vi "AbsImage_LFHelper_PIXIS_v0.1.vi"() -> ()   [LabVIEW 2012]
doc: "Take a single PixelFly exposure and display the result as an intensity graph.This VI illustrates the basics of taking an exposure with the PixelFly camera. Use Ctrl-H to get help on any of the controls\n\nCopyright 2001, The Cooke Corporation."
uses:
  LabVIEW Data V4.10/Shared Libraries/Controls/FileName_Cluster.ctl
  IMAQdx_AbsImage_Flea3_v4.2_RbYb/Shared Libraries/Controls/FileInfo_Global.vi
  <vilib>/Analysis/NI_AALBase.lvlib
panel:
  out "CycleDone":bool
  out "frame count":i64
  out "Loop":i32=3
  out "Status":string="Running..."
  in  "stop":bool
  in  "Tab Control":enum32{"Setup", "Images", "Hardware status"}(tab)=enum."Images"
  in  "SPE File Path":path=path "C:/Users/Lab/Documents/LightField/LabviewTemp.spe"
  in  "Experiment":T1(ring)=enum."Sr"
  in  "Accept parameters from remote system":bool=TRUE
  in  "Bias (Amps)":dbl
  in  "Pinch Coil (Amps)":dbl=520.0
  in  "Expansion time (ms)":dbl=19.0
  in  "Trap min at 0 (MHz)":dbl=2.85
  in  "Detuning (Linewidths)":dbl
  in  "Racetrack (Amps)":dbl=540.0
  in  "Magnification":dbl=5.66
  in  "Image direction":enum16{"XY", "XZ"}(ring)
  in  "Imaging technique":enum16{"Absorption", "Fluorescence", "RawImage"}(ring)
  in  "File Parameters":T2={"Data Root"=path "C:/Experiment/Data", "Index"=20198, "Instrument"="PIXIS"} {"Index" format="%04d"}
  in  "Send data to Igor?":bool=TRUE
  out "Command to Igor":string="AutoRunV3(\"Dipole_Load_Sr_88\",\"C:\\\\Experiment\\\\Data\\\\2013\\\\October\\\\09\\\\PIXIS_09Oct2013_20197.ibw\") "
  out "Image note":string="Experiment=Sr\nCamera_ID=PIXIS\nImageType=Raw\nDataType=Absorption\nImageDirection=XY\nMagnification=5.660000E+0\nFileNumber=20197\n# Current Variables\n# \nplus_zman=-1.800000E+0\nminus_zman=-1.500000E+0\ncompensation=-1.500000E+0\nMOTcoils=-1.250000E+0\nx=1.000000E+0\n# Master Staging List\n# Line\tMarker\tOption\tHalt\t0       4       8      12      16      20    AO\tDelay\t\tPoints\t0\t\t1\t\t2\t\t3\t\t4\t\t5\t\t6\t\t7\t\t8\t\t9\t\t10\t\t11\t\t12\t\t13\t\t14\t\t15\t\tComment\n00\t\tRamp\t0 0 0 0 0 0 0 0 0 0 1 0 0 1 0 0 0 0 0 0 0 0 0 0\t.5\t0\tplus_zman\tminus_zman\tcompensation\tMOTcoils\t0\t0\t0\t0\t0\t0\t0\t0\t0\t0\t0\t0\twait\n01\t\tRamp\t0 0 0 0 0 0 0 0 0 0 1 0 0 1 0 0 0 0 0 0 0 0 0 0\t.0001\t0\tplus_zman\tminus_zman\tcompensation\tMOTcoils\t0\t0\t0\t0\t0\t0\t0\t0\tLineRamp(f, 2,10)\t0\t0\t0\timg 1\n02\t\tRamp\t0 0 0 0 0 0 0 0 0 0 1 0 0 1 0 0 0 0 0 0 0 0 0 0\t.75\t0\tplus_zman\tminus_zman\tcompensation\tMOTcoils\t0\t0\t0\t0\t0\t0\t0\t0\t5\t0\t0\t0\ttransmit\n03\t\tRamp\t0 0 0 0 0 0 0 0 0 0 1 0 0 1 0 0 0 0 0 0 0 0 0 0\t.0001\t0\tplus_zman\tminus_zman\tcompensation\tMOTcoils\t0\t0\t0\t0\t0\t0\t0\t0\tSinRamp(t,5,2,5,0)\t0\t0\t0\timg 2\n04\t\tRamp\t0 0 0 0 0 0 0 0 0 0 1 0 0 1 0 0 0 0 0 0 0 0 0 0\t.75\t0\tplus_zman\tminus_zman\tcompensation\tMOTcoils\t0\t0\t0\t0\t0\t0\t0\t0\t0\t0\t0\t0\ttransmit\n05\t\tRamp\t0 0 0 0 0 0 0 0 0 0 1 0 0 1 0 0 0 0 0 0 0 0 0 0\t.0001\t0\t-1.8\t-1.5\t-1.5\t-1.25\t0\t0\t0\t0\t0\t0\t0\t0\t0\t0\t0\t0\timg 3\n06\t\tRamp\t0 0 0 0 0 0 0 0 0 0 1 0 0 1 0 0 0 0 0 0 0 0 0 0\t.75\t0\t-1.8\t-1.5\t-1.5\t-1.25\t0\t0\t0\t0\t0\t0\t0\t0\t0\t0\t0\t0\ttransmit\n07\t\tRamp\t0 0 0 0 0 0 0 0 0 0 1 0 0 1 0 0 0 0 0 0 0 0 0 0\t.0001\t0\t-1.8\t-1.5\t-1.5\t-1.25\t0\t0\t0\t0\t0\t0\t0\t0\t0\t0\t0\t0\timg 4\n08\t\tRamp\t0 0 0 0 0 0 0 0 0 0 1 0 0 1 0 0 0 0 0 0 0 0 0 0\t.75\t0\t-1.8\t-1.5\t-1.5\t-1.25\t0\t0\t0\t0\t0\t0\t0\t0\t0\t0\t0\t0\ttransmit\n# Slave Staging List\n# Line\tMarker\tOption\tHalt\t0       4       8      12      16      20    AO\tDelay\t\tPoints\t0\t\t1\t\t2\t\t3\t\t4\t\t5\t\t6\t\t7\t\t8\t\t9\t\t10\t\t11\t\t12\t\t13\t\t14\t\t15\t\tComment\n# SRS List\n# \n#\n# Evaporation\n\nDDS Table\r\n"
  in  "Igor Wave Name":string="Test_Img"
  in  "Save file to archive?":bool=TRUE
  in  "Quad [Amps]":dbl=540.0
  in  "Source of File Data":refnum<k21>="\\\\Control\\VariableLibrary\\Instruction String"
  in  "Bits to shift":i32
  out "SPE delete path":path=path "C:/Users/Lab/Documents/LightField/LabviewTemp.spe"
  in  "Source of Control Data":refnum<k21>="\\\\CONTROL\\VariableLibrary\\CycleDone"
  in  "Raw image to view":u16(ring)=3 items=["Clear", "Absorbtion", "Probe", "Background"]
  in  "Update Graphics":bool=TRUE
  out "Raw Image":u16[][](graph)
  out "Processed Image":sgl[][](graph)
  out "Histogram":cluster{"X Values":dbl[], dbl[]}(graph)={"X Values"=[222.6796875, 228.0390625, 233.3984375, 238.7578125, 244.1171875, 249.4765625, 254.8359375, 260.1953125, 265.5546875, 270.9140625, 276.2734375, 281.6328125, 286.9921875, 292.3515625, 297.7109375, 303.0703125, 308.4296875, 313.7890625, 319.1484375, 324.5078125, 329.8671875, 335.2265625, 340.5859375, 345.9453125, 351.3046875, 356.6640625, 362.0234375, 367.3828125, 372.7421875, 378.1015625, 383.4609375, 388.8203125, 394.1796875, 399.5390625, 404.8984375, 410.2578125, 415.6171875, 420.9765625, 426.3359375, 431.6953125, 437.0546875, 442.4140625, 447.7734375, 453.1328125, 458.4921875, 463.8515625, 469.2109375, 474.5703125, 479.9296875, 485.2890625, 490.6484375, 496.0078125, 501.3671875, 506.7265625, 512.0859375, 517.4453125, 522.8046875, 528.1640625, 533.5234375, 538.8828125, 544.2421875, 549.6015625, 554.9609375, 560.3203125], [0.0, 0.0, 0.47712125471966244, 0.9030899869919435, 1.3979400086720377, 1.7558748556724915, 1.9084850188786497, 2.0827853703164503, 2.2764618041732443, 2.250420002308894, 2.1702617153949575, 2.100370545117563, 1.6127838567197355, 1.4771212547196624, 0.9542425094393249, 0.6020599913279624, 0.0, 0.0, -inf, -inf, -inf, -inf, -inf, -inf, -inf, -inf, -inf, -inf, -inf, -inf, -inf, -inf, -inf, -inf, -inf, -inf, -inf, -inf, -inf, 0.6989700043360189, 1.0791812460476249, 1.9493900066449128, 2.3654879848909, 2.843855422623161, 3.4331295175804857, 3.7897921677306754, 4.159867847092567, 4.650734806320192, 4.868156391036818, 5.075243944428966, 5.299119245716857, 5.251701474421589, 5.273290705251327, 5.016795247263093, 4.796213427493061, 4.545406089684553, 4.046104787246039, 3.6663307443019684, 3.3366598234544202, 2.739572344450092, 2.374748346010104, 2.0, 1.255272505103306, 0.9542425094393249]}
  out "Images":u16[][][](array[numeric])
  out "SPE Load Error Out":errorcluster={"status"=FALSE, "code"=-1074360293, "source"="IMAQdx Get Image.vi"}
  out "DDE Error":errorcluster={"status"=TRUE, "code"=14012, "source"="DDE Execute: DMLERR_NOTPROCESSED"}
  in  "SPE Load Error In":errorcluster
  out "XML Parse Errors":string
  out "DataBlock Info":T3={"frame count"=4, "frame size"=2097152, "frame stride"=2097152, "N ROI"=1, "ROI widths"=[1024], "ROI heights"=[1024], "ROI sizes"=[2097152], "ROI strides"=[2097152]}
  out "Data Array Size":i32=1
  out "DS Error":errorcluster
  # "PIXIS Image Acquisition Helper v0.1"
  # "Experimental Paramaters"
  # "Sr: set to 0."
  # "In both techniques 3 images\nare aquired, but in Fluorescense\nthe 3rd is discarded"
  # "Sr: .663  is XZ\n     5.48 is XY"
  # "Obsolete: (now done with network variables)\nWhen paramaters are accepted from a remote system a DataSockets server\nmust be running on this machine (in start menu in National Instruments folder)"
  # "Output configuration"
  # "Input configuration"
  # "When the gain is 10 :  742 counts = Isat with 100 us pulse.  This is fine and\nis the point of highest SNR.  Linearized in software."
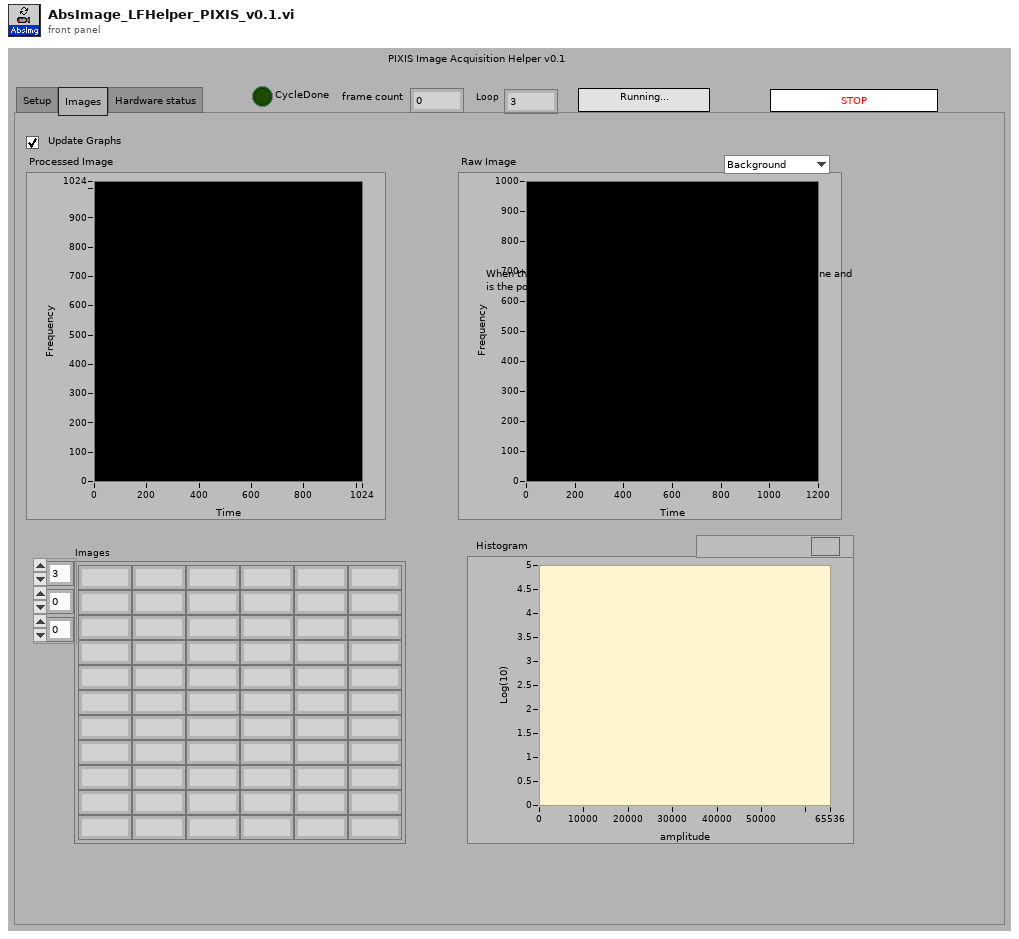
[diagram p1: front panel]
types:
  T1 = enum16{"Rubidium I", "Rubidium II", "RbLi", "RbYb", "Sr"}
  T2 = typedef "FileName_Cluster.ctl" = cluster{"Data Root":path, "Index":u32, "Instrument":string}
  T3 = cluster{"frame count":i64, "frame size":i64, "frame stride":i64, "N ROI":i64, "ROI widths":i64[], "ROI heights":i64[], "ROI sizes":i64[], "ROI strides":i64[]}
  T4 = cluster{"X Values":dbl[], "Histogram: h(x)":i32[]}
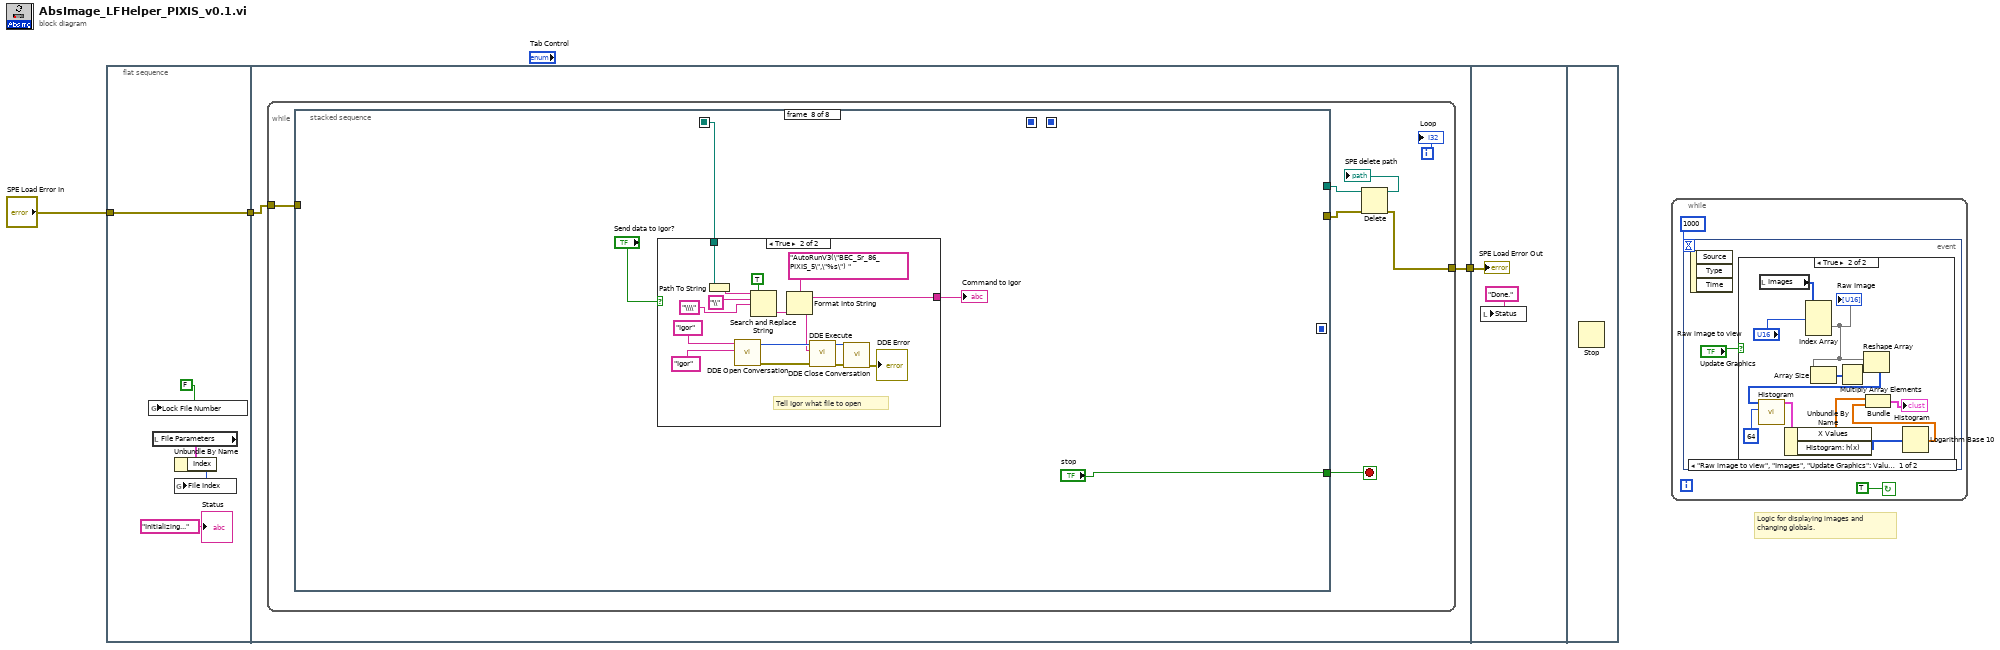
[diagram p0: block diagram]
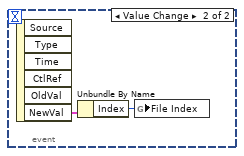
[diagram p3: hidden frame]
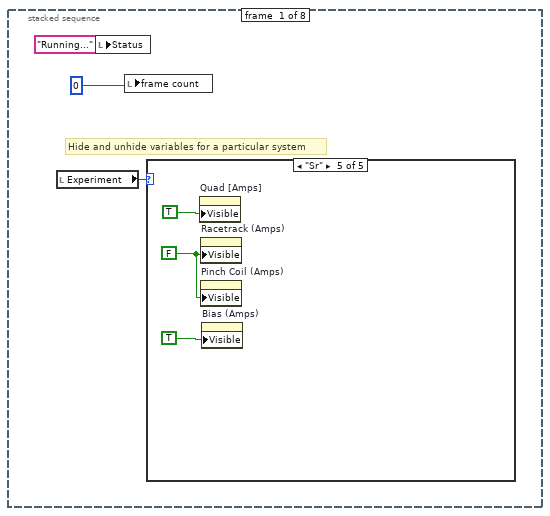
[diagram p4: hidden frame]
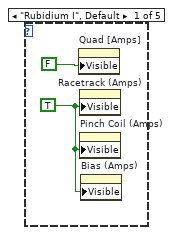
[diagram p5: hidden frame]
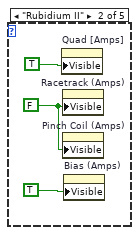
[diagram p6: hidden frame]
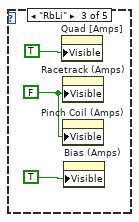
[diagram p7: hidden frame]
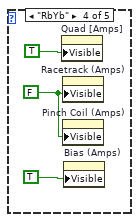
[diagram p8: hidden frame]
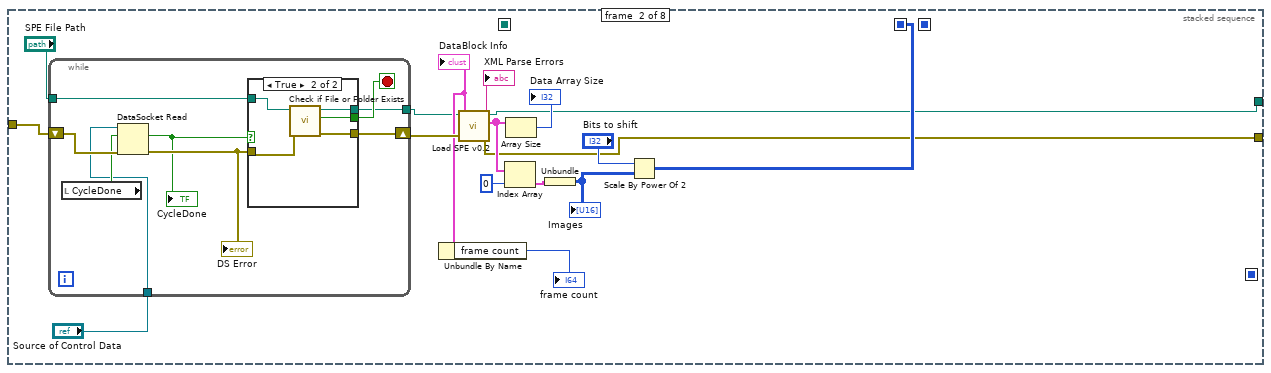
[diagram p9: hidden frame]
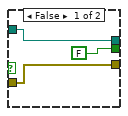
[diagram p10: hidden frame]
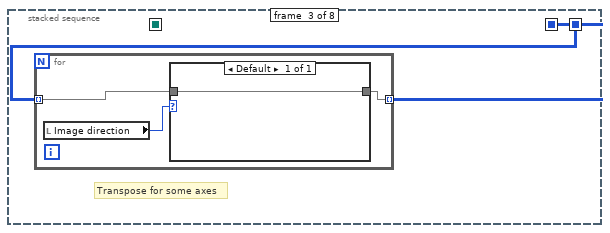
[diagram p11: hidden frame]
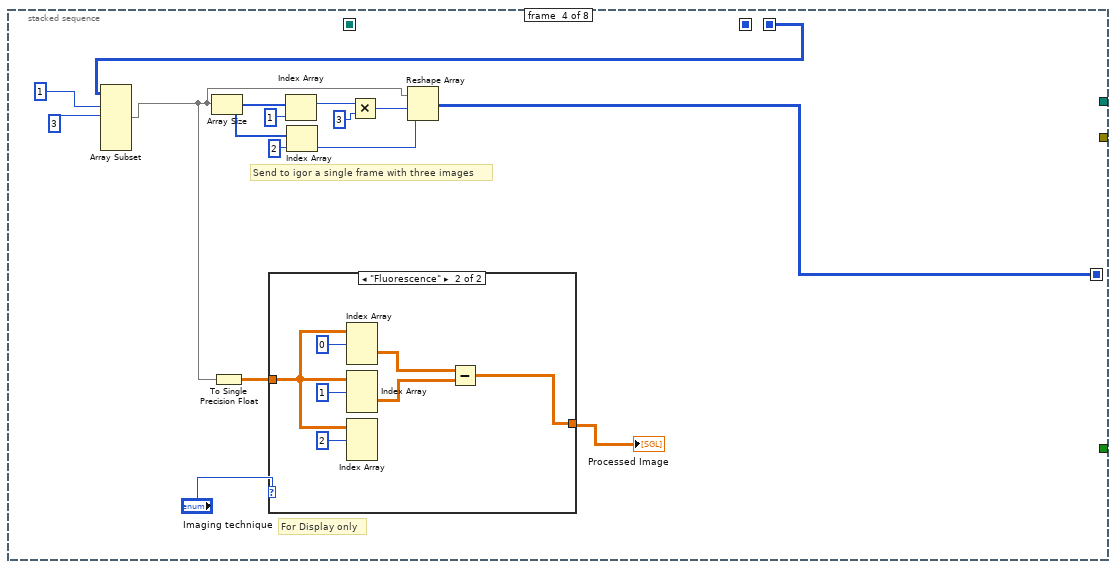
[diagram p12: hidden frame]
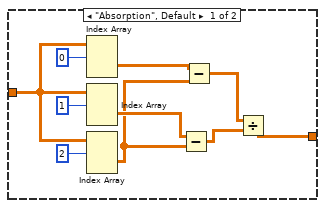
[diagram p13: hidden frame]
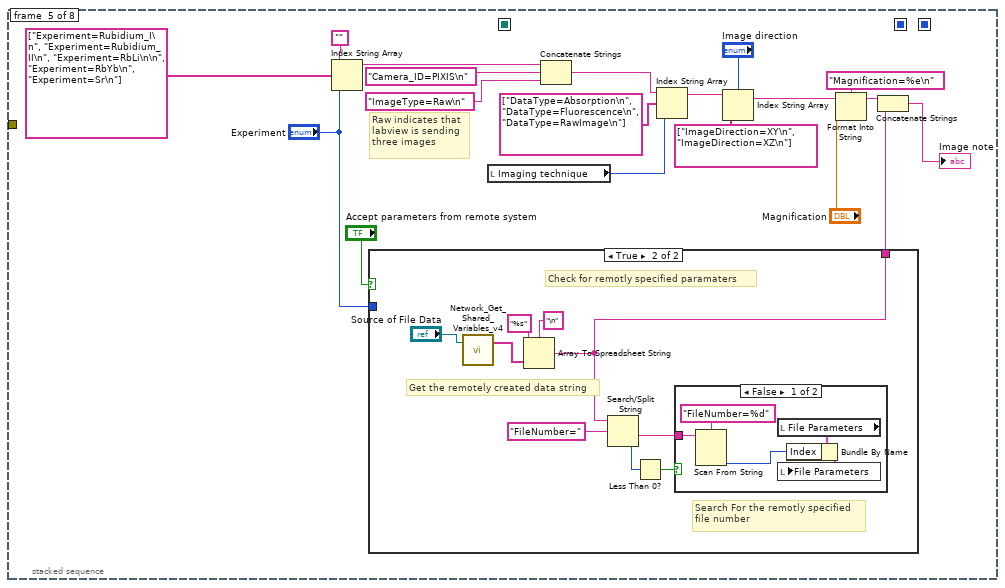
[diagram p14: hidden frame]
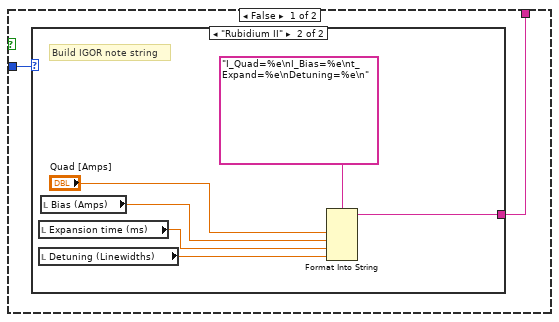
[diagram p15: hidden frame]
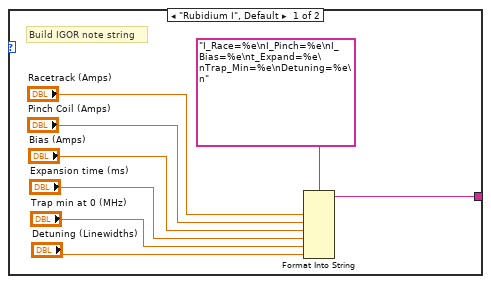
[diagram p16: hidden frame]
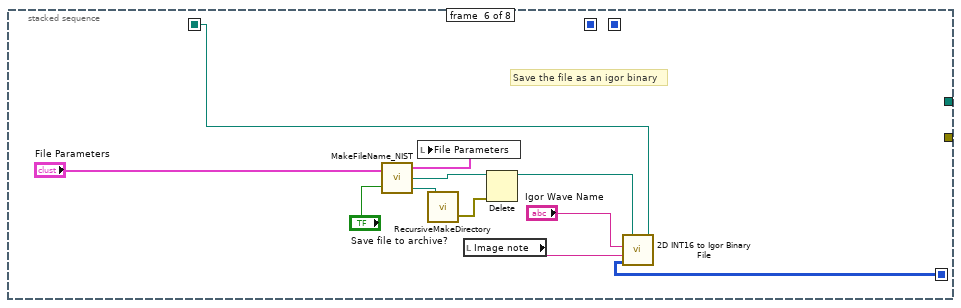
[diagram p18: hidden frame]
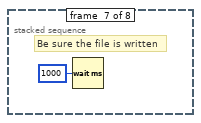
[diagram p19: hidden frame]
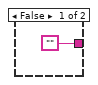
[diagram p20: hidden frame]
diagram:
  # "Logic for displaying images and\nchanging globals."
  n1 = flat-sequence {
    tunnel: "SPE Load Error In" -> [w4]
    tunnel: [w4] -> w2
    tunnel: w2 -> [w10]
    tunnel: [w9] -> w1
    tunnel: w1 -> [w188]
    frame #0 {
      n2 = global write "FileInfo_Global.vi" "Lock File Number"(FALSE) -> ()
      n3 = local read "File Parameters"() -> (w5:T2)
      n4 = Unbundle By Name(w5) -> ("Index"=w6:u32)
      n5 = global write "FileInfo_Global.vi" "File Index"(w6) -> ()
      "Status" <- "Initializing..."
    }
    frame #1 {
      n6 = while {
        tunnel: w10 -> [w15]
        tunnel: [w12] -> w9
        i -> [w17]
        stop <- w16 stop-if-true
        n7 = stacked-sequence {
          seq-local: [_ _ _ w87 _ _ _ _] -> [_ _ _ _ _ w160 _ _]
          seq-local: [_ _ _ _ _ w156 _ _] -> [_ _ _ _ _ _ _ w170]
          seq-local: [_ w41 _ _ _ _ _ _] -> [_ _ w70 _ _ _ _ _]
          seq-local: [_ _ w69 _ _ _ _ _] -> [_ _ _ w78 _ _ _ _]
          tunnel: [_ _ _ _ _ _ _ "stop"] -> w16
          tunnel: w15 -> [_ w49 _ _ _ _ _ _]
          tunnel: [_ w40 _ _ _ _ _ _] -> w14
          tunnel: [_ w39 _ _ _ _ _ _] -> w13
          frame #0 {
            # "Hide and unhide variables for a particular system"
            n8 = local read "Experiment"() -> (w19:T1)
            n9 = local write "Status"("Running...") -> ()
            n10 = local write "frame count"(i64 0) -> ()
            n11 = case shown="\"Sr\"" w19 {
              frame "Rubidium I", Default {
                w21 = TRUE
                n12 = property on="Quad [Amps]" class="DigNum (strict)"("Visible"=FALSE) -> ()  [unwired: 2 in, 2 out]
                n13 = property on="Racetrack (Amps)" class="DigNum (strict)"("Visible"=w21) -> ()  [unwired: 2 in, 2 out]
                n14 = property on="Pinch Coil (Amps)" class="DigNum (strict)"("Visible"=w21) -> ()  [unwired: 2 in, 2 out]
                n15 = property on="Bias (Amps)" class="DigNum (strict)"("Visible"=w21) -> ()  [unwired: 2 in, 2 out]
              }
              frame "Rubidium II" {
                w24 = FALSE
                n16 = property on="Quad [Amps]" class="DigNum (strict)"("Visible"=TRUE) -> ()  [unwired: 2 in, 2 out]
                n17 = property on="Racetrack (Amps)" class="DigNum (strict)"("Visible"=w24) -> ()  [unwired: 2 in, 2 out]
                n18 = property on="Pinch Coil (Amps)" class="DigNum (strict)"("Visible"=w24) -> ()  [unwired: 2 in, 2 out]
                n19 = property on="Bias (Amps)" class="DigNum (strict)"("Visible"=TRUE) -> ()  [unwired: 2 in, 2 out]
              }
              frame "RbLi" {
                w27 = FALSE
                n20 = property on="Quad [Amps]" class="DigNum (strict)"("Visible"=TRUE) -> ()  [unwired: 2 in, 2 out]
                n21 = property on="Racetrack (Amps)" class="DigNum (strict)"("Visible"=w27) -> ()  [unwired: 2 in, 2 out]
                n22 = property on="Pinch Coil (Amps)" class="DigNum (strict)"("Visible"=w27) -> ()  [unwired: 2 in, 2 out]
                n23 = property on="Bias (Amps)" class="DigNum (strict)"("Visible"=TRUE) -> ()  [unwired: 2 in, 2 out]
              }
              frame "RbYb" {
                w30 = FALSE
                n24 = property on="Quad [Amps]" class="DigNum (strict)"("Visible"=TRUE) -> ()  [unwired: 2 in, 2 out]
                n25 = property on="Racetrack (Amps)" class="DigNum (strict)"("Visible"=w30) -> ()  [unwired: 2 in, 2 out]
                n26 = property on="Pinch Coil (Amps)" class="DigNum (strict)"("Visible"=w30) -> ()  [unwired: 2 in, 2 out]
                n27 = property on="Bias (Amps)" class="DigNum (strict)"("Visible"=TRUE) -> ()  [unwired: 2 in, 2 out]
              }
              frame "Sr" {
                w33 = FALSE
                n28 = property on="Quad [Amps]" class="DigNum (strict)"("Visible"=TRUE) -> ()  [unwired: 2 in, 2 out]
                n29 = property on="Racetrack (Amps)" class="DigNum (strict)"("Visible"=w33) -> ()  [unwired: 2 in, 2 out]
                n30 = property on="Pinch Coil (Amps)" class="DigNum (strict)"("Visible"=w33) -> ()  [unwired: 2 in, 2 out]
                n31 = property on="Bias (Amps)" class="DigNum (strict)"("Visible"=TRUE) -> ()  [unwired: 2 in, 2 out]
              }
            }
          }
          frame #1 {
            n32 = while {
              tunnel: "SPE File Path" -> [w60]
              shift-right: [w59] -> w48
              shift-left: w49 -> [w56]
              tunnel: [w57] -> w36
              tunnel: "Source of Control Data" -> [w52]
              stop <- w58 stop-if-true
              n33 = local read "CycleDone"() -> (w55:bool)
              n34 = DataSocket Read(8:w56, 10:w55, 11:w52) -> (0:w54:errorcluster, 2:w53:bool)  [unwired: 2 in, 5 out]
              "CycleDone" <- w53
              "DS Error" <- w54
              n35 = case shown="True" w53 {
                tunnel: w60 -> [w63 w68]
                tunnel: [w62 w67] -> w59
                tunnel: [FALSE ("file or folder exists?") w66] -> w58
                tunnel: [w63 w65] -> w57
                tunnel: w54 -> [w62 w64]
                frame False {
                }
                frame True {
                  n36 = call <vilib>:"Check if File or Folder Exists.vi"("error in (no error)"=w64, "path"=w68) -> ("error out"=w67:errorcluster, "file or folder exists?"=w66:bool, "dup path"=w65:path)  [unwired: 7 in]
                }
              }
            }
            n37 = call "Load SPE v0.2.vi"("Error In"=w48, "File Path In"=w36) -> ("Error Out"=w39:errorcluster, "DataBlock Info"=w38:T3, "Output Stack"=w45:cluster{u16[][][]}[], "File Path Out"=w40:path, "Parse Errors"=→"XML Parse Errors":string)  [unwired: 5 in]
            "DataBlock Info" <- w38
            n38 = Unbundle By Name(w38) -> ("frame count"=→"frame count":i64)
            n39 = Index Array(array=w45, index=0) -> (element=w43:cluster{u16[][][]})
            n40 = Array Size(array=w45) -> (size(s)=→"Data Array Size":i32)
            n41 = Unbundle(w43) -> (w42:u16[][][])
            "Images" <- w42
            n42 = Scale By Power Of 2(n="Bits to shift", x=w42) -> (x*2^n=w41:u16[][][])
          }
          frame #2 {
            # "Transpose for some axes"
            n43 = for {
              tunnel: w70 -> [w72] mode=indexing
              tunnel: [w71] -> w69 mode=indexing
              n44 = local read "Image direction"() -> (w73:enum16{"XY", "XZ"})
              n45 = case shown="Default" w73 {
                tunnel: w72 -> [w74]
                tunnel: [w74] -> w71
                frame Default {
                }
              }
            }
          }
          frame #3 {
            # "Send to igor a single frame with three images"
            # "For Display only"
            n46 = Array Subset(array=w78, index (dim 0)=1 ("index"), length (dim 0)=3 ("length")) -> (w75:u16[][][])  [unwired: 4 in]
            n47 = Array Size(array=w75) -> (size(s)=w83:i32[])
            n48 = To Single Precision Float(number=w75) -> (single precision float=w84:sgl[][][])
            n49 = case shown="\"Fluorescence\"" "Imaging technique" {
              tunnel: [w96 w102] -> w88
              tunnel: w84 -> [w95 w103]
              frame "Absorption", Default {
                n50 = Index Array(array=w95, index (dim 0)=0 ("Number of buffers")) -> (element=w94:sgl[][])  [unwired: 2 in]
                n51 = Index Array(array=w95, index (dim 0)=1 ("Number of buffers")) -> (element=w93:sgl[][])  [unwired: 2 in]
                n52 = Index Array(array=w95, index (dim 0)=2 ("Number of buffers")) -> (element=w92:sgl[][])  [unwired: 2 in]
                n53 = Subtract(x=w93, y=w92) -> (x-y=w91:sgl[][])
                n54 = Subtract(x=w94, y=w92) -> (x-y=w90:sgl[][])
                n55 = Divide(x=w90, y=w91) -> (x/y=w96:sgl[][])
              }
              frame "Fluorescence" {
                n56 = Index Array(array=w103, index (dim 0)=0 ("Number of buffers")) -> (element=w101:sgl[][])  [unwired: 2 in]
                n57 = Index Array(array=w103, index (dim 0)=1 ("Number of buffers")) -> (element=w100:sgl[][])  [unwired: 2 in]
                n58 = Index Array(array=w103, index (dim 0)=2 ("Number of buffers")) -> ()  [unwired: 2 in, 1 out]
                n59 = Subtract(x=w101, y=w100) -> (x-y=w102:sgl[][])
              }
            }
            "Processed Image" <- w88
            n60 = Index Array(array=w83, index=1 ("Number of buffers")) -> (element=w80:i32)
            n61 = Index Array(array=w83, index=2 ("Number of buffers")) -> (element=w79:i32)
            n62 = Multiply(x=w80, y=3 ("Number of buffers")) -> (x*y=w85:i32)
            n63 = Reshape Array(w75, w85, w79) -> (w87:u16[][])
          }
          frame #4 {
            # "Raw indicates that\nlabview is sending\nthree images"
            n64 = Index String Array(1:"Experiment", 2:string[] ["Experiment=Rubidium_I\n", "Experiment=Rubidium_II\n", "Experiment=RbLi\n\n", "Experiment=RbYb\n", "Experiment=Sr\n"], 3:"") -> (0:w111:string)
            n65 = case shown="True" "Accept parameters from remote system" {
              tunnel: [w127 w143] -> w117
              tunnel: "Experiment" -> [w126 _]
              frame False {
                n66 = case shown="\"Rubidium II\"" w126 {
                  tunnel: [w128 w139] -> w127
                  frame "Rubidium I", Default {
                    # "Build IGOR note string"
                    n67 = Format Into String(format string="I_Race=%e\nI_Pinch=%e\nI_Bias=%e\nt_Expand=%e\nTrap_Min=%e\nDetuning=%e\n", "Racetrack (Amps)", "Pinch Coil (Amps)", "Bias (Amps)", "Expansion time (ms)", "Trap min at 0 (MHz)", "Detuning (Linewidths)") -> (resulting string=w128:string)  [unwired: 2 in, 1 out]
                  }
                  frame "Rubidium II" {
                    # "Build IGOR note string"
                    n68 = local read "Expansion time (ms)"() -> (w137:dbl)
                    n69 = local read "Detuning (Linewidths)"() -> (w136:dbl)
                    n70 = local read "Bias (Amps)"() -> (w138:dbl)
                    n71 = Format Into String(format string="I_Quad=%e\nI_Bias=%e\nt_Expand=%e\nDetuning=%e\n", "Quad [Amps]", w138, w137, w136) -> (resulting string=w139:string)  [unwired: 2 in, 1 out]
                  }
                }
              }
              frame True {
                # "Check for remotly specified paramaters"
                # "Get the remotely created data string"
                # "Search For the remotly specified\nfile number"
                n72 = call "Network_Get_Shared_Variables_v4.vi"("Source of Data"="Source of File Data") -> ("Igor Instruction String"=w150:string[])  [unwired: 1 in, 1 out]
                n73 = Array To Spreadsheet String(delimiter (Tab)="\n", array=w150, 3:"%s") -> (spreadsheet string=w143:string)
                n74 = Search/Split String(string=w143, search string/char (-)="FileNumber=") -> (match + rest of string=w146:string, offset of match=w145:i32)  [unwired: 2 out]
                n75 = Less Than 0?(x=w145) -> (x < 0?=w144:bool)
                n76 = case shown="False" w144 {
                  tunnel: w146 -> [w155 _]
                  frame False {
                    n77 = Scan From String(format string="FileNumber=%d", input string=w155) -> (output 1=w151:i32)  [unwired: 2 in, 4 out]
                    n78 = local read "File Parameters"() -> (w153:T2)
                    n79 = Bundle By Name(cluster=w153, "Index"=w151) -> (w152:T2)
                    n80 = local write "File Parameters"(w152) -> ()
                  }
                  frame True {
                  }
                }
              }
            }
            n81 = local read "Imaging technique"() -> (w122:enum16{"Absorption", "Fluorescence", "RawImage"})
            n82 = Concatenate Strings(w111, "Camera_ID=PIXIS\n", "ImageType=Raw\n") -> (w112:string)
            n83 = Index String Array(1:w122, 2:string[] ["DataType=Absorption\n", "DataType=Fluorescence\n", "DataType=RawImage\n"], 3:w112) -> (0:w123:string)
            n84 = Index String Array(1:"Image direction", 2:string[] ["ImageDirection=XY\n", "ImageDirection=XZ\n"], 3:w123) -> (0:w125:string)
            n85 = Format Into String(format string="Magnification=%e\n", initial string=w125, "Magnification") -> (resulting string=w119:string)  [unwired: 1 in, 1 out]
            n86 = Concatenate Strings(w119, w117) -> (→"Image note":string)
          }
          frame #5 {
            # "Save the file as an igor binary"
            n87 = call "MakeFileName_NIST.vi"("File Parameters"="File Parameters", "Save permanent file?"="Save file to archive?") -> ("New file parameters."=w162:T2, "Path to File"=w164:path, "path"=w163:path)
            n88 = local write "File Parameters"(w162) -> ()
            n89 = call "RecursiveMakeDirectory.vi"("Directory to create"=w163) -> ("error out"=w166:errorcluster)  [unwired: 1 in, 1 out]
            n90 = local read "Image note"() -> (w159:string)
            n91 = Delete(path (use dialog)=w164, error in=w166) -> (deleted path=w157:path)  [unwired: 5 out]
            n92 = call "2D INT16 to Igor Binary File.vi"("Wave Data (I16)"=w160, "Wave Note (\"\")"=w159, "WaveName"="Igor Wave Name", "Path (default: dialog)"=w157) -> ("Path chosen"=w156:path)
          }
          frame #6 {
            # "Be sure the file is written"
            n93 = Wait (ms)(milliseconds to wait=u32 1000) -> ()  [unwired: 1 out]
          }
          frame #7 {
            n94 = case shown="True" "Send data to Igor?" {
              tunnel: w170 -> [_ w179]
              tunnel: ["" w178] -> w169
              frame False {
              }
              frame True {
                # "Tell Igor what file to open"
                n95 = Path To String(path=w179) -> (string=w176:string)
                n96 = call <vilib>:"DDE Open Conversation.vi"("topic"="Igor", "service"="Igor") -> ("error out"=w183:errorcluster, "conversation refnum"=w181:u32)  [unwired: 1 in, 5 out]
                n97 = Search and Replace String(replace all?=TRUE, input string=w176, search string="\\", replace string="\\\\") -> (result string=w177:string)  [unwired: 1 in, 6 out]
                n98 = Format Into String(format string="AutoRunV3(\"BEC_Sr_86_PIXIS_5\",\"%s\") ", w177) -> (resulting string=w178:string)  [unwired: 2 in, 1 out]
                n99 = call <vilib>:"DDE Execute.vi"("error in (no error)"=w183, "command"=w178, "conversation refnum in"=w181) -> ("error out"=w182:errorcluster, "conversation refnum out"=w180:u32)  [unwired: 5 out]
                n100 = call <vilib>:"DDE Close Conversation.vi"("error in (no error)"=w182, "conversation refnum"=w180) -> ("error out"=→"DDE Error":errorcluster)  [unwired: 7 out]
              }
            }
            "Command to Igor" <- w169
          }
        }
        n101 = Delete(path (use dialog)=w14, error in=w13) -> (deleted path=→"SPE delete path":path, error out=w12:errorcluster)  [unwired: 3 in, 1 out]
        "Loop" <- w17
      }
    }
    frame #2 {
      n102 = local write "Status"("Done.") -> ()
      "SPE Load Error Out" <- w188
    }
    frame #3 {
      n103 = Stop() -> ()  [unwired: 1 out]
    }
  }
  n104 = while {
    stop <- TRUE continue-if-true
    n105 = event shown="[0] \"Raw image to view\", \"Images\", \"Update Graphics\": Value Change;  Timeout" {
      selector: _ -> [_ _]
      dyn-events: _ -> [_ _]
      timeout: 1000 -> [_ _]
      event "Raw image to view", "Images", "Update Graphics": Value Change; Timeout {
        n106 = event-data() -> ()  [unwired: 4 out]
        n107 = case shown="True" "Update Graphics" {
          frame False {
          }
          frame True {
            n108 = local read "Images"() -> (w204:u16[][][])
            n109 = Index Array(array=w204, index (dim 0)="Raw image to view") -> (element=w202:u16[][])  [unwired: 2 in]
            "Raw Image" <- w202
            n110 = Array Size(array=w202) -> (size(s)=w201:i32[])
            n111 = Multiply Array Elements(1:w201) -> (0:w200:i32)
            n112 = Reshape Array(w202, w200) -> (w198:u16[])
            n113 = call <vilib>:"Histogram.vi"("intervals"=64, "X"=w198) -> ("Histogram Graph"=w197:T4)  [unwired: 9 out]
            n114 = Unbundle By Name(w197) -> ("X Values"=w195:dbl[], "Histogram: h(x)"=w196:i32[])
            n115 = Logarithm Base 10(1:w196) -> (0:w194:dbl[])
            n116 = Bundle("X Values"=w195, w194) -> (→"Histogram":cluster{"X Values":dbl[], dbl[]})  [unwired: 1 out]
          }
        }
      }
      event Value Change {
        n117 = event-data() -> ("NewVal"=w205:T2)  [unwired: 6 out]
        n118 = Unbundle By Name(w205) -> ("Index"=w206:u32)
        n119 = global write "FileInfo_Global.vi" "File Index"(w206) -> ()
      }
    }
  }
